vi "SaccadeAnalyser - Main.vi"(8 "error in (no error)":errorcluster, 11 "Data IN":T3={"Impulse Positions"=[{"Start"=5471, "End"=5813, "Impulse Plane"=enum."Yaw", "Impulse Direction +ve?"=FALSE, "Time offset"=0, "Amplitude offset"=0.0}, {"Start"=6974, "End"=7325, "Impulse Plane"=enum."Yaw", "Impulse Direction +ve?"=TRUE, "Time offset"=0, "Amplitude offset"=0.0}, {"Start"=7641, "End"=7980, "Impulse Plane"=enum."Yaw", "Impulse Direction +ve?"=FALSE, "Time offset"=0, "Amplitude offset"=0.0}, {"Start"=9060, "End"=9400, "Impulse Plane"=enum."Yaw", "Impulse Direction +ve?"=FALSE, "Time offset"=0, "Amplitude offset"=0.0}, {"Start"=9938, "End"=10282, "Impulse Plane"=enum."Yaw", "Impulse Direction +ve?"=FALSE, "Time offset"=0, "Amplitude offset"=0.0}, {"Start"=10800, "End"=11142, "Impulse Plane"=enum."Yaw", "Impulse Direction +ve?"=FALSE, "Time offset"=0, "Amplitude offset"=0.0}, {"Start"=11602, "End"=11942, "Impulse Plane"=enum."Yaw", "Impulse Direction +ve?"=TRUE, "Time offset"=0, "Amplitude offset"=0.0}, {"Start"=12449, "End"=12790, "Impulse Plane"=enum."Yaw", "Impulse Direction +ve?"=TRUE, "Time offset"=0, "Amplitude offset"=0.0}, {"Start"=13310, "End"=13653, "Impulse Plane"=enum."Yaw", "Impulse Direction +ve?"=TRUE, "Time offset"=0, "Amplitude offset"=0.0}, {"Start"=14191, "End"=14535, "Impulse Plane"=enum."Yaw", "Impulse Direction +ve?"=TRUE, "Time offset"=0, "Amplitude offset"=0.0}, {"Start"=15040, "End"=15380, "Impulse Plane"=enum."Yaw", "Impulse Direction +ve?"=FALSE, "Time offset"=0, "Amplitude offset"=0.0}, {"Start"=16780, "End"=17124, "Impulse Plane"=enum."Yaw", "Impulse Direction +ve?"=TRUE, "Time offset"=0, "Amplitude offset"=0.0}, {"Start"=17572, "End"=17913, "Impulse Plane"=enum."Yaw", "Impulse Direction +ve?"=FALSE, "Time offset"=0, "Amplitude offset"=0.0}, {"Start"=18369, "End"=18713, "Impulse Plane"=enum."Yaw", "Impulse Direction +ve?"=FALSE, "Time offset"=0, "Amplitude offset"=0.0}, {"Start"=19174, "End"=19519, "Impulse Plane"=enum."Yaw", "Impulse Direction +ve?"=FALSE, "Time offset"=0, "Amplitude offset"=0.0}, {"Start"=19928, "End"=20270, "Impulse Plane"=enum."Yaw", "Impulse Direction +ve?"=TRUE, "Time offset"=0, "Amplitude offset"=0.0}, {"Start"=20762, "End"=21121, "Impulse Plane"=enum."Yaw", "Impulse Direction +ve?"=FALSE, "Time offset"=0, "Amplitude offset"=0.0}, {"Start"=21554, "End"=21888, "Impulse Plane"=enum."Yaw", "Impulse Direction +ve?"=FALSE, "Time offset"=0, "Amplitude offset"=0.0}, {"Start"=22293, "End"=22639, "Impulse Plane"=enum."Yaw", "Impulse Direction +ve?"=TRUE, "Time offset"=0, "Amplitude offset"=0.0}, {"Start"=23109, "End"=23464, "Impulse Plane"=enum."Yaw", "Impulse Direction +ve?"=TRUE, "Time offset"=0, "Amplitude offset"=0.0}, {"Start"=23868, "End"=24215, "Impulse Plane"=enum."Yaw", "Impulse Direction +ve?"=TRUE, "Time offset"=0, "Amplitude offset"=0.0}, {"Start"=24643, "End"=24992, "Impulse Plane"=enum."Yaw", "Impulse Direction +ve?"=FALSE, "Time offset"=0, "Amplitude offset"=0.0}, {"Start"=25685, "End"=26023, "Impulse Plane"=enum."Yaw", "Impulse Direction +ve?"=FALSE, "Time offset"=0, "Amplitude offset"=0.0}, {"Start"=26431, "End"=26768, "Impulse Plane"=enum."Yaw", "Impulse Direction +ve?"=FALSE, "Time offset"=0, "Amplitude offset"=0.0}, {"Start"=27251, "End"=27595, "Impulse Plane"=enum."Yaw", "Impulse Direction +ve?"=FALSE, "Time offset"=0, "Amplitude offset"=0.0}, {"Start"=28832, "End"=29180, "Impulse Plane"=enum."Yaw", "Impulse Direction +ve?"=TRUE, "Time offset"=0, "Amplitude offset"=0.0}, {"Start"=31028, "End"=31383, "Impulse Plane"=enum."LARP", "Impulse Direction +ve?"=FALSE, "Time offset"=0, "Amplitude offset"=0.0}, {"Start"=32603, "End"=32936, "Impulse Plane"=enum."LARP", "Impulse Direction +ve?"=TRUE, "Time offset"=0, "Amplitude offset"=0.0}, {"Start"=33445, "End"=33779, "Impulse Plane"=enum."LARP", "Impulse Direction +ve?"=TRUE, "Time offset"=0, "Amplitude offset"=0.0}, {"Start"=34276, "End"=34629, "Impulse Plane"=enum."LARP", "Impulse Direction +ve?"=FALSE, "Time offset"=0, "Amplitude offset"=0.0}, {"Start"=35114, "End"=35460, "Impulse Plane"=enum."LARP", "Impulse Direction +ve?"=FALSE, "Time offset"=0, "Amplitude offset"=0.0}, {"Start"=35981, "End"=36324, "Impulse Plane"=enum."LARP", "Impulse Direction +ve?"=TRUE, "Time offset"=0, "Amplitude offset"=0.0}, {"Start"=36920, "End"=37249, "Impulse Plane"=enum."LARP", "Impulse Direction +ve?"=TRUE, "Time offset"=0, "Amplitude offset"=0.0}, {"Start"=37988, "End"=38322, "Impulse Plane"=enum."LARP", "Impulse Direction +ve?"=TRUE, "Time offset"=0, "Amplitude offset"=0.0}, {"Start"=38964, "End"=39324, "Impulse Plane"=enum."LARP", "Impulse Direction +ve?"=FALSE, "Time offset"=0, "Amplitude offset"=0.0}, {"Start"=39948, "End"=40284, "Impulse Plane"=enum."LARP", "Impulse Direction +ve?"=TRUE, "Time offset"=0, "Amplitude offset"=0.0}, {"Start"=40958, "End"=41293, "Impulse Plane"=enum."LARP", "Impulse Direction +ve?"=TRUE, "Time offset"=0, "Amplitude offset"=0.0}, {"Start"=41899, "End"=42229, "Impulse Plane"=enum."LARP", "Impulse Direction +ve?"=TRUE, "Time offset"=0, "Amplitude offset"=0.0}, {"Start"=42801, "End"=43154, "Impulse Plane"=enum."LARP", "Impulse Direction +ve?"=FALSE, "Time offset"=0, "Amplitude offset"=0.0}, {"Start"=43641, "End"=43980, "Impulse Plane"=enum."LARP", "Impulse Direction +ve?"=TRUE, "Time offset"=0, "Amplitude offset"=0.0}, {"Start"=44466, "End"=44821, "Impulse Plane"=enum."LARP", "Impulse Direction +ve?"=FALSE, "Time offset"=0, "Amplitude offset"=0.0}, {"Start"=45388, "End"=45722, "Impulse Plane"=enum."LARP", "Impulse Direction +ve?"=TRUE, "Time offset"=0, "Amplitude offset"=0.0}, {"Start"=46149, "End"=46510, "Impulse Plane"=enum."LARP", "Impulse Direction +ve?"=FALSE, "Time offset"=0, "Amplitude offset"=0.0}, {"Start"=47874, "End"=48206, "Impulse Plane"=enum."LARP", "Impulse Direction +ve?"=TRUE, "Time offset"=0, "Amplitude offset"=0.0}, {"Start"=50143, "End"=50479, "Impulse Plane"=enum."RALP", "Impulse Direction +ve?"=TRUE, "Time offset"=0, "Amplitude offset"=0.0}, {"Start"=50976, "End"=51310, "Impulse Plane"=enum."RALP", "Impulse Direction +ve?"=FALSE, "Time offset"=0, "Amplitude offset"=0.0}, {"Start"=51892, "End"=52226, "Impulse Plane"=enum."RALP", "Impulse Direction +ve?"=FALSE, "Time offset"=0, "Amplitude offset"=0.0}, {"Start"=52839, "End"=53171, "Impulse Plane"=enum."RALP", "Impulse Direction +ve?"=FALSE, "Time offset"=0, "Amplitude offset"=0.0}, {"Start"=53676, "End"=54012, "Impulse Plane"=enum."RALP", "Impulse Direction +ve?"=TRUE, "Time offset"=0, "Amplitude offset"=0.0}, {"Start"=54530, "End"=54877, "Impulse Plane"=enum."RALP", "Impulse Direction +ve?"=FALSE, "Time offset"=0, "Amplitude offset"=0.0}, {"Start"=55371, "End"=55711, "Impulse Plane"=enum."RALP", "Impulse Direction +ve?"=TRUE, "Time offset"=0, "Amplitude offset"=0.0}, {"Start"=56153, "End"=56482, "Impulse Plane"=enum."RALP", "Impulse Direction +ve?"=FALSE, "Time offset"=0, "Amplitude offset"=0.0}, {"Start"=57053, "End"=57390, "Impulse Plane"=enum."RALP", "Impulse Direction +ve?"=FALSE, "Time offset"=0, "Amplitude offset"=0.0}, {"Start"=57954, "End"=58292, "Impulse Plane"=enum."RALP", "Impulse Direction +ve?"=FALSE, "Time offset"=0, "Amplitude offset"=0.0}, {"Start"=58794, "End"=59130, "Impulse Plane"=enum."RALP", "Impulse Direction +ve?"=TRUE, "Time offset"=0, "Amplitude offset"=0.0}, {"Start"=59587, "End"=59931, "Impulse Plane"=enum."RALP", "Impulse Direction +ve?"=TRUE, "Time offset"=0, "Amplitude offset"=0.0}, {"Start"=60399, "End"=60744, "Impulse Plane"=enum."RALP", "Impulse Direction +ve?"=FALSE, "Time offset"=0, "Amplitude offset"=0.0}, {"Start"=61218, "End"=61559, "Impulse Plane"=enum."RALP", "Impulse Direction +ve?"=FALSE, "Time offset"=0, "Amplitude offset"=0.0}, {"Start"=62100, "End"=62442, "Impulse Plane"=enum."RALP", "Impulse Direction +ve?"=FALSE, "Time offset"=0, "Amplitude offset"=0.0}, {"Start"=62989, "End"=63322, "Impulse Plane"=enum."RALP", "Impulse Direction +ve?"=FALSE, "Time offset"=0, "Amplitude offset"=0.0}, {"Start"=63787, "End"=64136, "Impulse Plane"=enum."RALP", "Impulse Direction +ve?"=TRUE, "Time offset"=0, "Amplitude offset"=0.0}, {"Start"=64603, "End"=64953, "Impulse Plane"=enum."RALP", "Impulse Direction +ve?"=FALSE, "Time offset"=0, "Amplitude offset"=0.0}, {"Start"=65462, "End"=65795, "Impulse Plane"=enum."RALP", "Impulse Direction +ve?"=FALSE, "Time offset"=0, "Amplitude offset"=0.0}, {"Start"=66308, "End"=66645, "Impulse Plane"=enum."RALP", "Impulse Direction +ve?"=FALSE, "Time offset"=0, "Amplitude offset"=0.0}, {"Start"=67052, "End"=67402, "Impulse Plane"=enum."RALP", "Impulse Direction +ve?"=TRUE, "Time offset"=0, "Amplitude offset"=0.0}], "No. Imp"=15, "Parameter Time Series"=[{"time offset"=0.0, "Offset"=0.0, "Gain"=1.0, "inverse"=FALSE, "filter data"=FALSE, "dots"=FALSE, "interpolate"=FALSE, "List 1"=5, "Color Box"=6618880, "Boolean"=TRUE}, {"time offset"=0.0, "Offset"=0.0, "Gain"=1.0, "inverse"=FALSE, "filter data"=FALSE, "dots"=FALSE, "interpolate"=FALSE, "List 1"=6, "Color Box"=6618880, "Boolean"=FALSE}, {"time offset"=0.0, "Offset"=0.0, "Gain"=1.0, "inverse"=FALSE, "filter data"=FALSE, "dots"=FALSE, "interpolate"=FALSE, "List 1"=7, "Color Box"=6618880, "Boolean"=FALSE}, {"time offset"=0.0, "Offset"=0.0, "Gain"=1.0, "inverse"=FALSE, "filter data"=FALSE, "dots"=FALSE, "interpolate"=FALSE, "List 1"=13, "Color Box"=16777224, "Boolean"=TRUE}, {"time offset"=0.0, "Offset"=0.0, "Gain"=1.0, "inverse"=FALSE, "filter data"=FALSE, "dots"=FALSE, "interpolate"=FALSE, "List 1"=14, "Color Box"=16777224, "Boolean"=FALSE}, {"time offset"=0.0, "Offset"=0.0, "Gain"=1.0, "inverse"=FALSE, "filter data"=FALSE, "dots"=FALSE, "interpolate"=FALSE, "List 1"=15, "Color Box"=16777224, "Boolean"=FALSE}], "Parameter Impuls Series"=[{"Color"=6618880, "Visible"=TRUE, "Channel"=1, "Invert"=FALSE, "Desaccade"=FALSE, "Offset"=0.0, "Gain"=1.0}, {"Color"=6618880, "Visible"=FALSE, "Channel"=6, "Invert"=FALSE, "Desaccade"=FALSE, "Offset"=0.0, "Gain"=1.0}, {"Color"=6618880, "Visible"=FALSE, "Channel"=7, "Invert"=FALSE, "Desaccade"=FALSE, "Offset"=0.0, "Gain"=1.0}, {"Color"=16777224, "Visible"=TRUE, "Channel"=13, "Invert"=FALSE, "Desaccade"=FALSE, "Offset"=0.0, "Gain"=1.0}, {"Color"=16777224, "Visible"=FALSE, "Channel"=14, "Invert"=FALSE, "Desaccade"=FALSE, "Offset"=0.0, "Gain"=1.0}, {"Color"=16777224, "Visible"=FALSE, "Channel"=15, "Invert"=FALSE, "Desaccade"=FALSE, "Offset"=0.0, "Gain"=1.0}], "Experiment Parameters"={"Freq"=0.0, "Vel"=0, "Acc"=0, "Stimulus"="Head Impulse"}, "Autosort File"=refnum, "Data File"={"Data Channels"=array34x71049[2415666 elements], "Sample Rate"=500, "Channel List"=["Hz Position-in-Head", "Hz Velocity-in-Head", "Hy Position-in-Head", "Hy Velocity-in-Head", "Hx Position-in-Head", "Hx Velocity-in-Head", "Hl Velocity-in-Head", "Hr Velocity-in-Head", "Lx Position-in-Head", "Ly Position-in-Head", "Lz Position-in-Head", "Lx Velocity-in-Head", "Ly Velocity-in-Head", "Lz Velocity-in-Head", "Ll Velocity-in-Head", "Lr Velocity-in-Head", "Rx Position-in-Head", "Ry Position-in-Head", "Rz Position-in-Head", "Rx Velocity-in-Head", "Ry Velocity-in-Head", "Rz Velocity-in-Head", "Rl Velocity-in-Head", "Rr Velocity-in-Head", "Target on/off", "aux input 1", "aux input 2", " ", "", "", "", "Target Hor", "Target Ver", ""]}, "Experiment data path"=path "C:/Users/w.figtree/Desktop/Coils Data/3", "Image data path"=path "/Macintosh HD/Users/patrick/Studium/Diploma Thesis/Data Analysis", "LVS data path"=path "/Macintosh HD/Users/patrick/Studium/Diploma Thesis/Data Analysis", "Raw copy path"=path "/Macintosh HD/Users/patrick/Studium/Diploma Thesis/Data Analysis", "filename"="passive_lvs.lvs", "desaccading parameters"={"Tolerance"=3, "Acc Range"=7000.0, "Sample Rate"=500, "Impulse Plane 2"=enum."Yaw", "Impulse dir"=FALSE}, "Experiment Parameters 2"={"Subject"="SE Trial Short Term", "Strain"="", "Rotation plane"="", "Experimenter"=" ", "Trial"=0.0, "Time"=0.0}, "Excel"={"Excel._Application"=refnum, "Use Excel"=TRUE, "Worksheet SINE"=refnum, "Row SINE"=0, "Worksheet TRANS"=refnum, "Row TRANS"=0}, "Session Config File"=refnum, "Autosort Parameter Set"=4, "EMA Version"="EMA 2016a", "desacc "={"Threshold 1 [Acc]"=7000.0, "Threshold 2 [% of TH1]"=60, "tolerance"=3, "Search WD "=0.1, " always use TH2"=FALSE, "Range"=3.0, "Max time"=120.0, "Min time"=20.0, "Velocity Threshold"=150}, "Cycle Nr for Saccades"={"POS"=0, "NEG"=0}, "calibration name"="u_calibration_1_p00001s001_calib.mat", "Excel"=refnum} {"Parameter Time Series"."time offset" format="%.3f"; "Parameter Time Series"."Gain" format="%.1f"; "Parameter Time Series"."Offset" format="%.1f"; "Parameter Time Series"."List 1" items=["Motor-Pos", "Motor-Vel", "Lx Position-in-Head", "Ly Position-in-Head", "Lz Position-in-Head", "Lx Velocity-in-Head", "Ly Velocity-in-Head", "Lz Velocity-in-Head", "Ll Velocity-in-Head", "Lr Velocity-in-Head", "Lx Accel-in-Head", "Ly Accel-in-Head", "Lz Accel-in-Head", "Rx Position-in-Head", "Ry Position-in-Head", "Rz Position-in-Head", "Rx Velocity-in-Head", "Ry Velocity-in-Head", "Rz Velocity-in-Head", "Rl Velocity-in-Head", "Rr Velocity-in-Head", "Rx Accel-in-Head", "Ry Accel-in-Head", "Rz Accel-in-Head", "Global Trigger", "", "", ""]; "Parameter Impuls Series"."Gain" format="%.1f"; "Parameter Impuls Series"."Offset" format="%.1f"}) -> (0 "error out":errorcluster, 3 "Data OUT":T3={"Impulse Positions"=[{"Start"=5471, "End"=5813, "Impulse Plane"=enum."Yaw", "Impulse Direction +ve?"=FALSE, "Time offset"=0, "Amplitude offset"=0.0}, {"Start"=6974, "End"=7325, "Impulse Plane"=enum."Yaw", "Impulse Direction +ve?"=TRUE, "Time offset"=0, "Amplitude offset"=0.0}, {"Start"=7641, "End"=7980, "Impulse Plane"=enum."Yaw", "Impulse Direction +ve?"=FALSE, "Time offset"=0, "Amplitude offset"=0.0}, {"Start"=9060, "End"=9400, "Impulse Plane"=enum."Yaw", "Impulse Direction +ve?"=FALSE, "Time offset"=0, "Amplitude offset"=0.0}, {"Start"=9938, "End"=10282, "Impulse Plane"=enum."Yaw", "Impulse Direction +ve?"=FALSE, "Time offset"=0, "Amplitude offset"=0.0}, {"Start"=10800, "End"=11142, "Impulse Plane"=enum."Yaw", "Impulse Direction +ve?"=FALSE, "Time offset"=0, "Amplitude offset"=0.0}, {"Start"=11602, "End"=11942, "Impulse Plane"=enum."Yaw", "Impulse Direction +ve?"=TRUE, "Time offset"=0, "Amplitude offset"=0.0}, {"Start"=12449, "End"=12790, "Impulse Plane"=enum."Yaw", "Impulse Direction +ve?"=TRUE, "Time offset"=0, "Amplitude offset"=0.0}, {"Start"=13310, "End"=13653, "Impulse Plane"=enum."Yaw", "Impulse Direction +ve?"=TRUE, "Time offset"=0, "Amplitude offset"=0.0}, {"Start"=14191, "End"=14535, "Impulse Plane"=enum."Yaw", "Impulse Direction +ve?"=TRUE, "Time offset"=0, "Amplitude offset"=0.0}, {"Start"=15040, "End"=15380, "Impulse Plane"=enum."Yaw", "Impulse Direction +ve?"=FALSE, "Time offset"=0, "Amplitude offset"=0.0}, {"Start"=16780, "End"=17124, "Impulse Plane"=enum."Yaw", "Impulse Direction +ve?"=TRUE, "Time offset"=0, "Amplitude offset"=0.0}, {"Start"=17572, "End"=17913, "Impulse Plane"=enum."Yaw", "Impulse Direction +ve?"=FALSE, "Time offset"=0, "Amplitude offset"=0.0}, {"Start"=18369, "End"=18713, "Impulse Plane"=enum."Yaw", "Impulse Direction +ve?"=FALSE, "Time offset"=0, "Amplitude offset"=0.0}, {"Start"=19174, "End"=19519, "Impulse Plane"=enum."Yaw", "Impulse Direction +ve?"=FALSE, "Time offset"=0, "Amplitude offset"=0.0}, {"Start"=19928, "End"=20270, "Impulse Plane"=enum."Yaw", "Impulse Direction +ve?"=TRUE, "Time offset"=0, "Amplitude offset"=0.0}, {"Start"=20762, "End"=21121, "Impulse Plane"=enum."Yaw", "Impulse Direction +ve?"=FALSE, "Time offset"=0, "Amplitude offset"=0.0}, {"Start"=21554, "End"=21888, "Impulse Plane"=enum."Yaw", "Impulse Direction +ve?"=FALSE, "Time offset"=0, "Amplitude offset"=0.0}, {"Start"=22293, "End"=22639, "Impulse Plane"=enum."Yaw", "Impulse Direction +ve?"=TRUE, "Time offset"=0, "Amplitude offset"=0.0}, {"Start"=23109, "End"=23464, "Impulse Plane"=enum."Yaw", "Impulse Direction +ve?"=TRUE, "Time offset"=0, "Amplitude offset"=0.0}, {"Start"=23868, "End"=24215, "Impulse Plane"=enum."Yaw", "Impulse Direction +ve?"=TRUE, "Time offset"=0, "Amplitude offset"=0.0}, {"Start"=24643, "End"=24992, "Impulse Plane"=enum."Yaw", "Impulse Direction +ve?"=FALSE, "Time offset"=0, "Amplitude offset"=0.0}, {"Start"=25685, "End"=26023, "Impulse Plane"=enum."Yaw", "Impulse Direction +ve?"=FALSE, "Time offset"=0, "Amplitude offset"=0.0}, {"Start"=26431, "End"=26768, "Impulse Plane"=enum."Yaw", "Impulse Direction +ve?"=FALSE, "Time offset"=0, "Amplitude offset"=0.0}, {"Start"=27251, "End"=27595, "Impulse Plane"=enum."Yaw", "Impulse Direction +ve?"=FALSE, "Time offset"=0, "Amplitude offset"=0.0}, {"Start"=28832, "End"=29180, "Impulse Plane"=enum."Yaw", "Impulse Direction +ve?"=TRUE, "Time offset"=0, "Amplitude offset"=0.0}, {"Start"=31028, "End"=31383, "Impulse Plane"=enum."LARP", "Impulse Direction +ve?"=FALSE, "Time offset"=0, "Amplitude offset"=0.0}, {"Start"=32603, "End"=32936, "Impulse Plane"=enum."LARP", "Impulse Direction +ve?"=TRUE, "Time offset"=0, "Amplitude offset"=0.0}, {"Start"=33445, "End"=33779, "Impulse Plane"=enum."LARP", "Impulse Direction +ve?"=TRUE, "Time offset"=0, "Amplitude offset"=0.0}, {"Start"=34276, "End"=34629, "Impulse Plane"=enum."LARP", "Impulse Direction +ve?"=FALSE, "Time offset"=0, "Amplitude offset"=0.0}, {"Start"=35114, "End"=35460, "Impulse Plane"=enum."LARP", "Impulse Direction +ve?"=FALSE, "Time offset"=0, "Amplitude offset"=0.0}, {"Start"=35981, "End"=36324, "Impulse Plane"=enum."LARP", "Impulse Direction +ve?"=TRUE, "Time offset"=0, "Amplitude offset"=0.0}, {"Start"=36920, "End"=37249, "Impulse Plane"=enum."LARP", "Impulse Direction +ve?"=TRUE, "Time offset"=0, "Amplitude offset"=0.0}, {"Start"=37988, "End"=38322, "Impulse Plane"=enum."LARP", "Impulse Direction +ve?"=TRUE, "Time offset"=0, "Amplitude offset"=0.0}, {"Start"=38964, "End"=39324, "Impulse Plane"=enum."LARP", "Impulse Direction +ve?"=FALSE, "Time offset"=0, "Amplitude offset"=0.0}, {"Start"=39948, "End"=40284, "Impulse Plane"=enum."LARP", "Impulse Direction +ve?"=TRUE, "Time offset"=0, "Amplitude offset"=0.0}, {"Start"=40958, "End"=41293, "Impulse Plane"=enum."LARP", "Impulse Direction +ve?"=TRUE, "Time offset"=0, "Amplitude offset"=0.0}, {"Start"=41899, "End"=42229, "Impulse Plane"=enum."LARP", "Impulse Direction +ve?"=TRUE, "Time offset"=0, "Amplitude offset"=0.0}, {"Start"=42801, "End"=43154, "Impulse Plane"=enum."LARP", "Impulse Direction +ve?"=FALSE, "Time offset"=0, "Amplitude offset"=0.0}, {"Start"=43641, "End"=43980, "Impulse Plane"=enum."LARP", "Impulse Direction +ve?"=TRUE, "Time offset"=0, "Amplitude offset"=0.0}, {"Start"=44466, "End"=44821, "Impulse Plane"=enum."LARP", "Impulse Direction +ve?"=FALSE, "Time offset"=0, "Amplitude offset"=0.0}, {"Start"=45388, "End"=45722, "Impulse Plane"=enum."LARP", "Impulse Direction +ve?"=TRUE, "Time offset"=0, "Amplitude offset"=0.0}, {"Start"=46149, "End"=46510, "Impulse Plane"=enum."LARP", "Impulse Direction +ve?"=FALSE, "Time offset"=0, "Amplitude offset"=0.0}, {"Start"=47874, "End"=48206, "Impulse Plane"=enum."LARP", "Impulse Direction +ve?"=TRUE, "Time offset"=0, "Amplitude offset"=0.0}, {"Start"=50143, "End"=50479, "Impulse Plane"=enum."RALP", "Impulse Direction +ve?"=TRUE, "Time offset"=0, "Amplitude offset"=0.0}, {"Start"=50976, "End"=51310, "Impulse Plane"=enum."RALP", "Impulse Direction +ve?"=FALSE, "Time offset"=0, "Amplitude offset"=0.0}, {"Start"=51892, "End"=52226, "Impulse Plane"=enum."RALP", "Impulse Direction +ve?"=FALSE, "Time offset"=0, "Amplitude offset"=0.0}, {"Start"=52839, "End"=53171, "Impulse Plane"=enum."RALP", "Impulse Direction +ve?"=FALSE, "Time offset"=0, "Amplitude offset"=0.0}, {"Start"=53676, "End"=54012, "Impulse Plane"=enum."RALP", "Impulse Direction +ve?"=TRUE, "Time offset"=0, "Amplitude offset"=0.0}, {"Start"=54530, "End"=54877, "Impulse Plane"=enum."RALP", "Impulse Direction +ve?"=FALSE, "Time offset"=0, "Amplitude offset"=0.0}, {"Start"=55371, "End"=55711, "Impulse Plane"=enum."RALP", "Impulse Direction +ve?"=TRUE, "Time offset"=0, "Amplitude offset"=0.0}, {"Start" (continued)
348.00000000000006, 350.00000000000006, 352.0, 354.0, 356.0, 358.0, 360.0, 362.0, 364.0, 366.0, 368.0, 370.0, 372.0, 374.0, 376.0, 378.0, 380.0, 382.0, 384.0, 386.0, 388.0, 390.0, 392.0, 394.0, 396.0, 398.0, 400.0, 402.0, 404.0, 406.0, 408.00000000000006, 410.00000000000006, 412.00000000000006, 414.00000000000006, 416.00000000000006, 418.0, 420.0, 422.0, 424.0, 426.0, 428.0, 430.0, 432.0, 434.0, 436.0, 438.0, 440.0, 442.0, 444.0, 446.0, 448.0, 450.0, 452.0, 454.0, 456.0, 458.0, 460.0, 462.0, 464.0, 466.0, 468.0, 470.00000000000006, 472.00000000000006, 474.00000000000006, 476.00000000000006, 478.00000000000006, 480.0, 482.0, 484.0, 486.0, 488.0, 490.0, 492.0, 494.0, 496.0, 498.0, 500.0, 502.0, 504.0, 506.0, 508.0, 510.0, 512.0, 514.0, 516.0, 518.0, 520.0, 522.0, 524.0, 526.0, 528.0, 530.0, 532.0, 534.0, 536.0, 538.0, 540.0, 542.0, 544.0, 546.0, 548.0, 550.0, 552.0, 554.0, 556.0, 558.0, 560.0, 562.0, 564.0, 566.0000000000001, 568.0000000000001, 570.0000000000001, 572.0000000000001, 574.0000000000001, 576.0000000000001, 578.0, 580.0, 582.0, 584.0, 586.0, 588.0, 590.0, 592.0, 594.0, 596.0, 598.0, 600.0, 602.0, 604.0, 606.0, 608.0, 610.0, 612.0, 614.0, 616.0, 618.0, 620.0, 622.0, 624.0, 626.0, 628.0, 630.0, 632.0, 634.0, 636.0, 638.0, 640.0, 642.0, 644.0, 646.0, 648.0, 650.0, 652.0, 654.0, 656.0, 658.0, 660.0, 662.0, 664.0, 666.0, 668.0], [1.6412623886928461, 2.488406667081785, 3.365123168864116, 4.156616880738532, 4.75085582942973, 5.06490335878749, 5.053808814643649, 4.713139090397474, 4.0925434386517345, 3.290242896963189, 2.43515037437583, 1.6781217641249917, 1.1635496431665828, 0.9864296793452709, 1.180235476852614, 1.7114859425154592, 2.4744371835381784, 3.3166862324157336, 4.068053244773418, 4.571855262254786, 4.717935512445626, 4.471322569554048, 3.8823914357969773, 3.069171753226811, 2.1943776057199194, 1.4344586853401875, 0.9397401847742403, 0.794962980880807, 0.9981375355794779, 1.4710503667792916, 2.0863712171691433, 2.686898395386498, 3.1227358051509473, 3.2946962307348397, 3.1732475588931535, 2.804361527699513, 2.2956981744978275, 1.7900314505141175, 1.42692953316085, 1.3020747788309954, 1.4494016068634714, 1.838405181956439, 2.3825986617375516, 2.965951798657944, 3.4734284970527263, 3.8287918695664356, 4.012108804514213, 4.047283560147911, 3.999491745244875, 3.955158460466249, 3.9870582133024124, 4.1378964445923465, 4.408520454023579, 4.75549298900185, 5.111890647118412, 5.419396028197087, 5.647431277048132, 5.803513616303825, 5.92678393754562, 6.070153826744665, 6.2837111300879105, 6.586140082286999, 6.950425315566808, 7.311690478533821, 7.5827644200318005, 7.67358423433849, 7.526061395503863, 7.14964513037277, 6.620079202564641, 6.063521367121591, 5.632865638561892, 5.476714468996943, 5.709802112963681, 6.385763451719397, 7.493496230284357, 8.971571394319017, 10.730716169889899, 12.665145207631326, 14.670655223042601, 16.669326810859996, 18.61338452484305, 20.478864908485143, 22.26407749114619, 24.00501513248515, 25.774201718637634, 27.66923439037243, 29.81877838579065, 32.372663053764065, 35.46724273414959, 39.20392675196207, 43.637473382158525, 48.75440041008244, 54.46592863679897, 60.63447464624389, 67.10347569905883, 73.72784393285843, 80.41364283392565, 87.1340792847199, 93.93054404438162, 100.89548624809755, 108.13475549264363, 115.72745554399087, 123.69365392315169, 131.98244338979165, 140.46695833220696, 148.96807425002913, 157.30062018043574, 165.3115338815591, 172.89379698383186, 179.9937574177297, 186.62689397087115, 192.85490940111166, 198.7519431287235, 204.38769580178905, 209.80858013191778, 215.02340694228445, 219.99688066274842, 224.64453534320438, 228.8337243804808, 232.3917650442524, 235.1145486884668, 236.7844124344026, 237.19564216250276, 236.17763306267557, 233.60933694212392, 229.43074605080028, 223.64924203715537, 216.32777447124852, 207.57720576715838, 197.544163400661, 186.39150800505712, 174.2958395791465, 161.4389064642977, 148.00976204341347, 134.21942491509554, 120.29113696265378, 106.44540000887365, 92.8937258549432, 79.81441796587703, 67.33264310065499, 55.51198012119663, 44.346214854288846, 33.779147525587334, 23.7398666061357, 14.171925573773684, 5.056477983326053, -3.5700207127816803, -11.628354946023615, -19.013339866237544, -25.6144945132613, -31.370254724826765, -36.291457656813876, -40.44610405272022, -43.94867348925448, -46.94050846694606, -49.554968147900894, -51.888031919511775, -53.98227661746645, -55.832234891492874, -57.39751057797592, -58.61172757320207, -59.39987336652423, -59.705183952766234, -59.49839105656891, -58.75976549523697, -57.47293191795647, -55.63007799846697, -53.2286891974485, -50.265982937938674, -46.74909238868217, -42.71900745889994, -38.25438290911218, -33.471997535539295, -28.53873267246679, -23.65596408438708, -19.028304765987272, -14.849560925532767, -11.271067906618605, -8.358679233120373, -6.0914358991664255, -4.3723817407781915, -3.0350273228936224, -1.8790236179919102, -0.7185513325720461, 0.5880598132042536, 2.109059169750406, 3.8098678571783964, 5.568815970322758, 7.215075708354458, 8.564763930604585, 9.45408010350648, 9.772227593149788, 9.497048870403951, 8.697288642608306, 7.509197448833508, 6.108195992533471, 4.677923912440466, 3.3647623606416683, 2.261363870910838, 1.4141273989997263, 0.8064920564532745, 0.3660643001950259, -0.008534456940209267, -0.42666015412406466, -0.9897963196516617, -1.7763501027783164, -2.8295658526289635, -4.1566442932605785, -5.717161512956999, -7.421820689830833, -9.150862998561895, -10.764275755377005, -12.132967239480962, -13.171280438721674, -13.836847317205148, -14.14227066736528, -14.166658403818788, -14.030806026533261, -13.863331869808151, -13.772513904776838, -13.828356449097582, -14.044288763979562, -14.366146888556063, -14.708258100458004, -14.980434179245709, -15.100778556268507, -15.033599929059447, -14.796405196253835, -14.4306275771838, -13.992101005171094, -13.541401409357208, -13.107769188131574, -12.678867813295371, -12.216855233215579, -11.679810622080142, -11.04653585916903, -10.33113475273609, -9.584657895461758, -8.885364891766104, -8.316558236113421, -7.939071194327411, -7.776656136953683, -7.810841445087117, -7.981803490098784, -8.201561091907518, -8.3755128714246, -8.429718649479772, -8.330164090809332, -8.078531554224863, -7.705053331576598, -7.258807177583639, -6.796932054955323, -6.376300301186481, -6.0328720085710215, -5.779927198455345, -5.61963697268701, -5.543142802905564, -5.538491620382547, -5.590157631270944, -5.673104987023572, -5.762204881135559, -5.829832782947797, -5.843200500532499, -5.773720619590841, -5.600334959668404, -5.316363272159452, -4.934619526502251, -4.483547280679933, -4.008273273122242, -3.565424345032744, -3.219887723650805, -3.0535182774148275, -3.1494311743180123, -3.5766356591885984, -4.38434899329162, -5.569271417729928, -7.038075410780015, -8.577769843416434, -9.850303709444205, -10.436079719799327, -9.89643731331821, -7.860113468983564, -4.139867507193869, 1.1836393543016275, 7.714366955283603, 14.747407872743832, 21.37706522917261, 26.656315254909103, 29.755925905755753, 30.1306788554151, 27.65294175194612, 22.631211021641793, 15.742249750023644, 7.917552080655157, 0.16434731585808038, -6.624286177975039, -11.814424012090928, -15.105823184589445, -16.53122154971252, -16.40521618929207, -15.215912519074433, -13.498067256588318, -11.73103720824053, -10.260247547743777, -9.26796101646042, -8.795975610075459, -8.77712999429341, -9.073606487240632, -9.5295291414611, -10.006230337033722, -10.398872258897317, -10.639246694082344, -10.698219411303247, -10.586421763680784, -10.341649720559804, -10.027953619930862, -9.725044691054913, -9.506162365746166, -9.429712226242597, -9.522434491285136, -9.761751337091237, -10.091085510467888, -10.437683637255383, -10.717922902684379, -10.858280687531384, -10.824684977558002, -10.631198810003776, -10.319617968818825, -9.954440694355444, -9.617072487758644, -9.367129314375454, -9.231205642460829, -9.212725722385008, -9.278420052089581]}, {[0.0, 2.0, 4.0, 6.0, 8.0, 10.0, 12.0, 14.0, 16.0, 18.000000000000004, 20.0, 22.0, 24.0, 26.000000000000004, 28.0, 30.0, 32.0, 34.0, 36.00000000000001, 38.0, 40.0, 42.0, 44.0, 46.0, 48.0, 50.0, 52.00000000000001, 54.0, 56.0, 58.0, 60.0, 62.0, 64.0, 66.0, 68.0, 70.0, 72.00000000000001, 74.0, 76.0, 78.0, 80.0, 82.0, 84.0, 86.0, 88.0, 90.0, 92.0, 94.0, 96.0, 98.0, 100.0, 102.00000000000001, 104.00000000000001, 106.0, 108.0, 110.0, 112.0, 114.0, 116.0, 118.00000000000001, 120.0, 122.0, 124.0, 126.0, 128.0, 130.0, 132.0, 134.0, 136.0, 138.0, 140.0, 142.00000000000003, 144.00000000000003, 146.0, 148.0, 150.0, 152.0, 154.0, 156.0, 158.0, 160.0, 162.0, 164.0, 166.0, 168.0, 170.0, 172.0, 174.00000000000003, 176.0, 178.0, 180.0, 182.0, 184.0, 186.0, 188.0, 190.0, 192.0, 194.0, 196.0, 198.0, 200.0, 202.0, 204.00000000000003, 206.00000000000003, 208.00000000000003, 210.0, 212.0, 214.0, 216.0, 218.0, 220.0, 222.0, 224.0, 226.0, 228.0, 230.0, 232.0, 234.0, 236.00000000000003, 238.00000000000003, 240.0, 242.0, 244.0, 246.0, 248.0, 250.0, 252.0, 254.0, 256.0, 258.0, 260.0, 262.0, 264.0, 266.0, 268.0, 270.0, 272.0, 274.0, 276.0, 278.0, 280.0, 282.0, 284.00000000000006, 286.00000000000006, 288.00000000000006, 290.0, 292.0, 294.0, 296.0, 298.0, 300.0, 302.0, 304.0, 306.0, 308.0, 310.0, 312.0, 314.0, 316.0, 318.0, 320.0, 322.0, 324.0, 326.0, 328.0, 330.0, 332.0, 334.0, 336.0, 338.0, 340.0, 342.0, 344.0, 346.00000000000006, 348.00000000000006, 350.00000000000006, 352.0, 354.0, 356.0, 358.0, 360.0, 362.0, 364.0, 366.0, 368.0, 370.0, 372.0, 374.0, 376.0, 378.0, 380.0, 382.0, 384.0, 386.0, 388.0, 390.0, 392.0, 394.0, 396.0, 398.0, 400.0, 402.0, 404.0, 406.0, 408.00000000000006, 410.00000000000006, 412.00000000000006, 414.00000000000006, 416.00000000000006, 418.0, 420.0, 422.0, 424.0, 426.0, 428.0, 430.0, 432.0, 434.0, 436.0, 438.0, 440.0, 442.0, 444.0, 446.0, 448.0, 450.0, 452.0, 454.0, 456.0, 458.0, 460.0, 462.0, 464.0, 466.0, 468.0, 470.00000000000006, 472.00000000000006, 474.00000000000006, 476.00000000000006, 478.00000000000006, 480.0, 482.0, 484.0, 486.0, 488.0, 490.0, 492.0, 494.0, 496.0, 498.0, 500.0, 502.0, 504.0, 506.0, 508.0, 510.0, 512.0, 514.0, 516.0, 518.0, 520.0, 522.0, 524.0, 526.0, 528.0, 530.0, 532.0, 534.0, 536.0, 538.0, 540.0, 542.0, 544.0, 546.0, 548.0, 550.0, 552.0, 554.0, 556.0, 558.0, 560.0, 562.0, 564.0, 566.0000000000001, 568.0000000000001, 570.0000000000001, 572.0000000000001, 574.0000000000001, 576.0000000000001, 578.0, 580.0, 582.0, 584.0, 586.0, 588.0, 590.0, 592.0, 594.0, 596.0, 598.0, 600.0, 602.0, 604.0, 606.0, 608.0, 610.0, 612.0, 614.0, 616.0, 618.0, 620.0, 622.0, 624.0, 626.0, 628.0, 630.0, 632.0, 634.0, 636.0, 638.0, 640.0, 642.0, 644.0, 646.0, 648.0, 650.0, 652.0, 654.0, 656.0, 658.0, 660.0, 662.0, 664.0, 666.0, 668.0], [-2.385127960658771, -2.726105221825227, -3.2017163154721757, -3.7213434098385108, -4.174255040430188, -4.458116998446039, -4.508928104569913, -4.313198479768025, -3.9105487119132425, -3.385197002030652, -2.8449071240314376, -2.4043706466848818, -2.157289101497528, -2.141764850120099, -2.3402624181839173, -2.692973881118471, -3.110078773741787, -3.497415494679993, -3.776600199203538, -3.8999598541623426, -3.854652541340674, -3.664314054734446, -3.3888666444297546, -3.0990647162139706, -2.8536926262475375, -2.6955422407208918, -2.6494504692886904, -2.715900544738904, -2.86679938023335, -3.0617511454002146, -3.2690423068182675, -3.4596281848223747, -3.6108986359846593, -3.717005408369417, -3.783103680832566, -3.8225496430619588, -3.8527686594079604, -3.8926748543812195, -3.9564422558252854, -4.046430950993898, -4.158156048746607, -4.281470484657225, -4.40343578106908, -4.5207599281070525, -4.634350924735829, -4.74912760908919, -4.881892950319933, -5.043436179590222, -5.234377846792407, -5.451361870737253, -5.677046607762952, -5.881556056728986, -6.03281599658635, -6.105460273858494, -6.084037564832115, -5.97368022061706, -5.809541070429819, -5.646377745013693, -5.540514204264566, -5.5374385199329925, -5.665955086835687, -5.927240572210856, -6.290032433304866, -6.698630992356902, -7.086504225748463, -7.387368448104083, -7.557461147275539, -7.59578519894916, -7.537786002633627, -7.448216981706777, -7.41319991533299, -7.520816269667899, -7.845002175501264, -8.43254333314649, -9.290664134568463, -10.388535332685327, -11.671589052023261, -13.067697206440277, -14.500957493565274, -15.912938913552788, -17.272005169943764, -18.577123003381345, -19.860084056316595, -21.194293054279967, -22.685473611433544, -24.4466007401951, -26.591181312424595, -29.225001526429324, -32.42512246314817, -36.22889246952825, -40.63736676587909, -45.622447700031174, -51.13287094854823, -57.11207808430182, -63.51329519227872, -70.30923804067359, -77.49976733119409, -85.09806477794855, -93.12590802475953, -101.60314690210903, -110.51701081936082, -119.80442129525792, -129.34877121679443, -138.98660005151535, -148.51372057013347, -157.70583992929602, -166.35294863494013, -174.2918909706102, -181.41658578888007, -187.67617549749716, -193.08648108964564, -197.7167400793523, -201.6628130418782, -205.02490232592288, -207.88225032119723, -210.2778956143569, -212.20927936619466, -213.61862316077244, -214.395759695901, -214.39306122413842, -213.44879780765257, -211.40752300153142, -208.14201380426078, -203.5883115030676, -197.75067126692224, -190.6884283783521, -182.5088115899605, -173.34392807944948, -163.33441467025577, -152.60876437570636, -141.26133618963422, -129.3600582168661, -116.95170075293805, -104.08308023146986, -90.83025841506038, -77.29937326936988, -63.63072735470836, -50.00080585933101, -36.60324036194258, -23.62476252231884, -11.217841816749564, 0.5169434352554805, 11.528317357379581, 21.806535231717916, 31.366757098379242, 40.21982348498953, 48.35357657552993, 55.737152674237116, 62.31201490630476, 67.99639254899691, 72.72557568491479, 76.47306172824122, 79.24557885964782, 81.08482807307318, 82.06825826366631, 82.29069633811068, 81.8508799191022, 80.83956402685664, 79.32675101044643, 77.36630119801063, 75.00065508870736, 72.25820301176982, 69.16012237808943, 65.7311410256808, 61.99598762973978, 57.97483494061889, 53.6898904691194, 49.16564798711905, 44.42638014494089, 39.50013777598713, 34.424898564633764, 29.25600342219904, 24.065843116655746, 18.940920509590473, 13.982511658037549, 9.296645573897301, 4.982552538366974, 1.1206059290617745, -2.2465227025181616, -5.117430213269211, -7.529816192066621, -9.555244319809027, -11.27856962600759, -12.78169723244285, -14.134734095569694, -15.373855058942427, -16.485082074836733, -17.421593505364072, -18.115897082335806, -18.488897967004768, -18.469620062324523, -18.01341073329258, -17.121796125894015, -15.845002785634382, -14.268586714916196, -12.5010570739269, -10.664879730090789, -8.865982662077492, -7.177925211951897, -5.645485447149259, -4.270513746242997, -3.014226817631071, -1.815938408421637, -0.6079551018088818, 0.6760032862715288, 2.0836614411401104, 3.631907048404411, 5.3116346741018585, 7.076305435707779, 8.844289078542666, 10.522335647932897, 12.00889974695749, 13.216544996318536, 14.09741101904055, 14.632275295706151, 14.837204302419536, 14.77454242395562, 14.527692487872487, 14.182426601575992, 13.813282476334866, 13.472247270559645, 13.189734954219102, 12.963141561566047, 12.771809270578004, 12.597858343176283, 12.422379080284312, 12.235583160956958, 12.04171159231155, 11.846019596711827, 11.648842181496365, 11.443238087765362, 11.20797835883704, 10.91147635404771, 10.522539324015508, 10.022512942589275, 9.423386112935818, 8.771984604678996, 8.13307410709041, 7.5778691819411765, 7.170516234328703, 6.941934124949661, 6.879019304246361, 6.931238242232464, 7.01771903105549, 7.0462531570010585, 6.946389263331276, 6.685159238822836, 6.275204488650119, 5.774310099858705, 5.261407463844925, 4.8149232632157934, 4.4963531367125515, 4.333176300878805, 4.306708301429621, 4.366107055664725, 4.453133883712994, 4.510570698852731, 4.501373780597615, 4.417286187062055, 4.267958955851897, 4.077203284769039, 3.8682708822534817, 3.654627159077674, 3.4399891229883792, 3.2142110883596207, 2.968886813102668, 2.711770381625172, 2.464007610350329, 2.261589301356673, 2.1458333639809606, 2.152785360099868, 2.310642312680236, 2.613651194234296, 3.019189705126233, 3.471702032923214, 3.907344245033122, 4.2671826906709605, 4.510532123273797, 4.620013959521999, 4.609822695992307, 4.514284640495481, 4.373857034361924, 4.23355522883207, 4.126200935072816, 4.072582136394162, 4.0978779361915505, 4.220308319393676, 4.443022467476181, 4.762501782961454, 5.168325247959957, 5.628337072312796, 6.094117000338438, 6.51951332915382, 6.858261224934491, 7.075647732283527, 7.168544494716964, 7.16430364452585, 7.109757580336011, 7.061831471398985, 7.074000225552721, 7.176322525667028, 7.370395905692706, 7.633001485563749, 7.915864539351305, 8.163212139077464, 8.33822131554868, 8.42537860709589, 8.429853085142705, 8.385660309923217, 8.342206808058574, 8.339889945581069, 8.396359534255378, 8.505006099739214, 8.636617685808154, 8.744514359078337, 8.786747350376244, 8.739856604354475, 8.604836172865, 8.41629561936021, 8.228408189966942, 8.092656129513571, 8.050684268786991, 8.12141931806205, 8.28994416286302, 8.512644299567505, 8.728624555858673, 8.879695934957649, 8.918822790314413, 8.81791382933297, 8.580585678696401, 8.22804119195135, 7.794227519284796, 7.3311514098975525, 6.885218245896482]}]
  # "Saccade Detection:"
  # "Stimulus Detection:"
  # "Gain Window:"
  # "Impulse Window:"
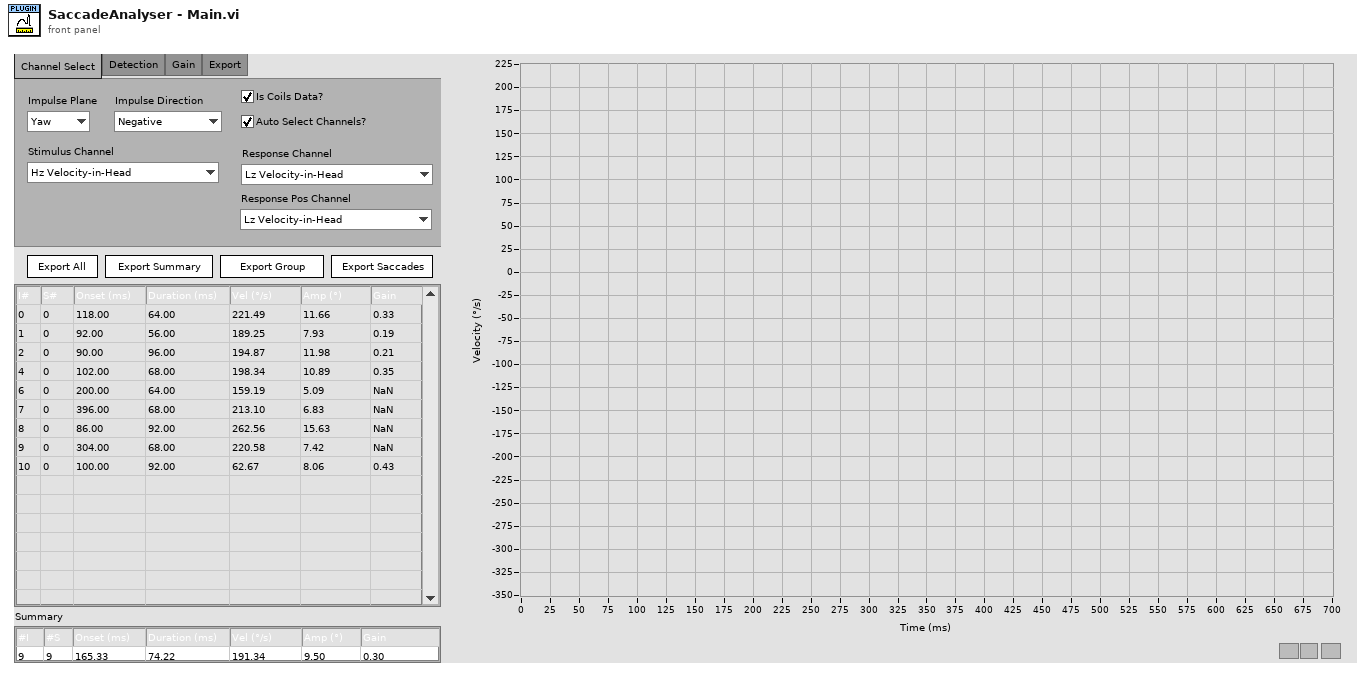
[diagram p1: front panel]
types:
  T1 = enum32{"Channel Select", "Detection", "Gain", "Export"}
  T2 = typedef "Saccade Analyser Impulse Plane.ctl" = enum16{"Other", "Yaw", "Pitch", "Roll", "LARP", "RALP"}
  T3 = typedef "core.lvlib/TD_Statemachine-Data.ctl" = cluster{"Impulse Positions":cluster{"Start":i32, "End":i32, "Impulse Plane":enum16{"Other", "Yaw", "Pitch", "Roll", "LARP", "RALP"}, "Impulse Direction +ve?":bool, "Time offset":i32, "Amplitude offset":dbl}[], "No. Imp":i32, "Parameter Time Series":T4, "Parameter Impuls Series":T5, "Experiment Parameters":cluster{"Freq":dbl, "Vel":i32, "Acc":i32, "Stimulus":string}, "Autosort File":refnum<file>, "Data File":cluster{"Data Channels":dbl[][], "Sample Rate":i32, "Channel List":string[]}, "Experiment data path":path, "Image data path":path, "LVS data path":path, "Raw copy path":path, "filename":string, "desaccading parameters":cluster{"Tolerance":i32, "Acc Range":dbl, "Sample Rate":i32, "Impulse Plane 2":enum16{"Other", "Yaw", "Pitch", "Roll", "LARP", "RALP"}, "Impulse dir":bool}, "Experiment Parameters 2":cluster{"Subject":string, "Strain":string, "Rotation plane":string, "Experimenter":string, "Trial":dbl, "Time":dbl}, "Excel":cluster{"Excel._Application":refnum<k7>, "Use Excel":bool, "Worksheet SINE":refnum<k7>, "Row SINE":i32, "Worksheet TRANS":refnum<k7>, "Row TRANS":i32}, "Session Config File":refnum<file>, "Autosort Parameter Set":i32, "EMA Version":string, "desacc ":cluster{"Threshold 1 [Acc]":dbl, "Threshold 2 [% of TH1]":i32, "tolerance":i32, "Search WD ":dbl, " always use TH2":bool, "Range":dbl, "Max time":dbl, "Min time":dbl, "Velocity Threshold":i32}, "Cycle Nr for Saccades":cluster{"POS":i32, "NEG":i32}, "calibration name":string, "Excel":refnum<class "Excel.lvclass">}
  T4 = typedef "core.lvlib/TD_Time Series.ctl" = cluster{"time offset":dbl, "Offset":dbl, "Gain":dbl, "inverse":bool, "filter data":bool, "dots":bool, "interpolate":bool, "List 1":u16, "Color Box":u32, "Boolean":bool}[]
  T5 = typedef "core.lvlib/TD_Impulse Parameter.ctl" = cluster{"Color":u32, "Visible":bool, "Channel":u16, "Invert":bool, "Desaccade":bool, "Offset":dbl, "Gain":dbl}[]
  T6 = typedef "Saccade Analyser Data.ctl" = cluster{"Impulse Data":refnum<data-value>, "Sample Rate (Hz)":dbl, "Num Impulses":i32, "Impulse Duration (samples)":i32, "Palette":T7, "Saccades":T8[], "Summary":T9, "Group Summary":T9[]}
  T7 = typedef "Saccade Analyser Palete Data.ctl" = cluster{"Stimulus":u32, "Response":u32, "Saccade":u32, "Excluded Saccade":u32, "Sibling Saccade":u32, "Selected Saccade":u32}